vi "HFRR ADV v040 new software.vi"() -> ()   [LabVIEW 2025] (continued)
  # "Move the carriage to the mechanical zero stop — no displacement applied. Before measuring, the sensor must be Preset. Once in position, tap Tare & Begin to zero the reference."
  # "Step 8 — POSITION MEASUREMENT"
  # "Measurement Checklist"
  # "Position the carriage at exactly this \nvalue using your reference gauge, then tap Confirm &\n Next."
  # "Stroked recorded!\n\nTap Confirm & Next  to review the calibration summary."
  # "Step 9 — CALIBRATION RESULT"
  # "Stroke Calibration Complete"
  # "Calibration completed successfully. The measured stroke length is within the acceptable tolerance range of the factory calibration value."
  # "Calibration failed. The measured stroke length differs from the factory calibration value by more than 20%. Please perform the calibration again."
  # "Step 1 — Ball Holder"
  # "Remove the ball holder by loosening and removing the center screw for Friction calibration."
  # "Step 2 — Disc Holder"
  # "Remove the disc holder by loosening and removing the opposing screws. Clean any fluid present in the disc holder."
  # "Step 3 — Calibration Head"
  # "Place the calibration holder in position and securely tighten the center screw."
  # "Step 4 — Calibration Holder"
  # "Place the calibration holder in position and tighten the two securing screws"
  # "Step 5 — Tare (Spring at Free Length)"
  # "Ensure the spring is at its contact (compressed) length — the micrometer head is in contact. Click Tare Sensor to zero the friction force baseline."
  # "Step 6 — Measure Friction Force"
  # "Run the Actual Test to measure Friction Force."
  # "Spring Constant: k = 1.000 N/mm\nSpring force |F| = k Ч d"
  # "Calibrates the ambient air temperature sensor."
  # "Calibrates the sample temperature sensor."
  # "Set B\n60 °C\nHigh-point calibration"
  # "Set A\n0 °C\nIce-point calibration"
  # "Set B\n60 °C\nHigh-point calibration"
  # "Set A\n0 °C\nIce-point calibration"
  # "Select Temperature Sensor"
  # "Choose which temperature sensor you are calibrating. Both use the same two-\npoint procedure: 0 °C (ice-point) and 60 °C (high-point)."
  # "Step 1 — Reference Instrument Setup"
  # "Connect a calibrated reference to the DUT port. This calibration performs two sets: one at 0 °C and one at 60 °C."
  # "Set A\n0 °C\nIce-point calibration"
  # "Set B\n60 °C\nHigh-point calibration"
  # "Allow the temperature bath to stabilise for at least 2 minutes at each set-point before recording the reading."
  # "Step 2 — Set A:  0 °C Calibration"
  # "Connect the  0 °C reference connector. Wait for the temperature to stabilise. Once stable, and click Record Point."
  # "Step 3 — Set A:  60 °C Calibration"
  # "Connect the  60 °C reference connector. Wait for the temperature to stabilise. Once stable, and click Record Point."
  # "Sample Temperature Calibration Complete"
  # "Sample Temperature Calibration PASSED\nMax deviation 0.200 °C — within ±0.5 °C tolerance. Two-point correction applied (0 °C & 60 °C)."
  # "Sample  Temperature Calibration Failed\nmeasured Sample Temperature differs from the factory calibration value"
  # "Step 1 — Reference Instrument Setup"
  # "Connect a calibrated reference to the DUT port. This calibration performs two sets: one at 0 °C and one at 60 °C."
  # "Set A\n0 °C\nIce-point calibration"
  # "Set B\n60 °C\nHigh-point calibration"
  # "Allow the temperature bath to stabilise for at least 2 minutes at each set-point before recording the reading."
  # "Step 2 — Set A:  0 °C Calibration"
  # "Connect the  0 °C reference connector. Wait for the temperature to stabilise. Once stable, and click Record Point."
  # "Step 3 — Set A:  60 °C Calibration"
  # "Connect the  60 °C reference connector. Wait for the temperature to stabilise. Once stable, and click Record Point."
  # "Air Temperature Calibration Complete"
  # "Air Temperature Calibration PASSED\nMax deviation 0.200 °C — within ±0.5 °C tolerance. Two-point correction applied (0 °C & 60 °C)."
  # "Air  Temperature Calibration Failed\nmeasured Sample Temperature differs from the factory calibration value"
  # "System Control Commands\nS;1 - Starts the full automation cycle (Runs Priming-humidify till 70RH sequence first, then switches to Maintenance).\nS;0 - Stops the system immediately and enters Standby mode (Safe State: All actuators OFF).\nM;1 - Skips the priming sequence and jumps directly to Maintenance mode (PID control).\nR;1 - Resets the logic state machine and clears all errors, returning to Standby.\nService Mode (Manual Control)\nX;1 - Enters Manual Service Mode. This disables all automatic logic, sensor safety checks, and timers.\nX;0 - Exits Manual Service Mode and returns to Standby (Safe State).\nActuator Commands (Only work after sending X;1)\nP;[0-255] - Sets the Pump PWM. Note that this is Active Low (0 = Max Flow, 255 = Pump OFF).\nF;I;[0-255] - Sets the Intake Fan speed (0 = OFF, 255 = Max Speed).\nF;O;[0-255] - Sets the Exhaust Fan speed (0 = OFF, 255 = Max Speed).\nD;1 - Turns the Dehumidifier Relay ON.\nD;0 - Turns the Dehumidifier Relay OFF."
  # "%RH"
  # "ISO : WS1.4"
  # "Start test and end test log--- done\nDisable heater ON and Humidity ON during the test --- done\ntemprature and ---done\nhumidity reach log\nauto start run true logic and log\nmanual start log once"
  # "Reference Fluid Information"
  # "Note:\nMake sure to place all images in the folder \"C:\\WinDucom\\im\" before clicking on \"Import Image.\""
  # "NOTE:\nPlace all the images in the path \"C:\\WinDucom\\im\" before clicking on Import Image"
  # "Wear Scar Measurements"
  # "Reference Fluid Information"
  # "Graph :"
types:
  T1 = enum32{"Home", "Dashboard", "Imaging", "Report", "Analysis", "About", "Test Setup", "Advance", "Calibration"}
  T2 = enum32{"HOME", "Test Setup", "Acquire", "Adv Scar", "Adv Scar Report", "Compare Files", "Calibration", "About", "Advance", "Mooha"}
  T3 = enum16{"ASTM D6079", "ISO 12156", "CEC F-096-A-06", "Custom"}
  T4 = enum32{"Dashboard 1", "Dashboard 2", "Dashboard 3"}
  T5 = enum32{"COF", "Friction", "ECR", "Temperature", "Stroke"}
  T6 = enum32{"Coefficient Of Friction", "Air Temperature", "Humidity", "Stroke", "Sample Temperature", "Electrical Contact Resistance", "Frequency", "Air Temp vs Rh"}
  T7 = enum32{"Main", "Stroke", "Friction", "Temperature"}
  T8 = enum32{"Stroke Calibration", "Friction Force Calibration", "Temperature Calibration", "Default"}
  T9 = enum32{"Step 1", "Step 2", "Step 3", "Step 4", "Step 5", "Step 6", "Step 7", "Step 8", "Step 9"}
  T10 = enum32{"Test Progress", "Stroke Points Completed"}
  T11 = enum32{"Page 1", "Page 2", "Page 3", "Page 4", "Page 5", "Page 6", "Page 7"}
  T12 = enum32{"Main", "Step 1", "Step 2", "Step 3", "Step 4", "Air Step 1", "Air Step 2", "Air Step 3", "Air Step 4"}
  T13 = enum32{"Air Temperature", "Sample Temperature", "Default"}
  T14 = enum32{"COMMUNICATION", "CALIBRATION", "Temp Variables", "Camera", "WO 2465 (1)", "WO 2465 (2)", "WO 2465 (3)"}
  T15 = typedef "Auto Start enum.ctl" = enum16{"Init", "Humidity & Temperature On", "Reach point", "Maintain Stage", "Start Stage", "close", "Exit"}
  T16 = typedef "imagedata.ctl" = cluster{"image type":i32, "image depth":i32, "image":u8[], "mask":u8[], "colors":u32[], "Rectangle":cluster{"left":i16, "top":i16, "right":i16, "bottom":i16}}
  T17 = enum32{"HOME", "Test Setup", "Acquire", "Compare Files", "Print Report", "About", "Advance", "Mooha"}
  T18 = cluster{"Read Heave and Surge":string, "Bytes at Heave Port":dbl, "Heave and Surge COM Port:":refnum<visa-resource-name>, "Com Port 2":refnum<visa-resource-name>, "Residual Due":string, "Heave COM Status 2":bool, "Heave COM Status":bool, "Port 2":bool, "Sway PPR":dbl, "Surge PPR":dbl, "Heave PPR":dbl, "Sway Pitch":dbl, "Surge Pitch":dbl, "Heave Pitch":dbl, "Sway Pulses/mm":dbl, "Surge Pulses/mm":dbl, "Heave Pulses/mm":dbl, "inner loop":dbl, "Read Heave and Surge 2":string, "String 36":string, "Write S":bool, "WriteCC1":string[], "Heave COM Loop":i32, "LastCom":string, "EXIT":bool, "Error Heave":errorcluster}
  T19 = enum8{"Enabled", "Disabled", "Disabled and Grayed Out"}
  T20 = cluster{"Read Uno":string, "Bytes at Heave Port":dbl, "UNO COM Port:":refnum<visa-resource-name>, "UNO COM Port: 2":refnum<visa-resource-name>, "Residual Due":string, "UNO COM Status 2":bool, "UNO COM Status":bool, "Port 2":bool, "Sway PPR":dbl, "Surge PPR":dbl, "Heave PPR":dbl, "Sway Pitch":dbl, "Surge Pitch":dbl, "Heave Pitch":dbl, "Sway Pulses/mm":dbl, "Surge Pulses/mm":dbl, "Heave Pulses/mm":dbl, "inner loop":dbl, "Read Heave and Surge 2":string, "String 36":string, "Write S":bool, "WriteCC1":string[], "Heave COM Loop":i32, "LastCom":string, "EXIT":bool, "Error Heave":errorcluster}
  T21 = enum32{"HOME", "Test Setup", "Acquire", "Adv Scar", "Adv Scar Report", "Compare Files", "About", "Advance", "Mooha"}
  T22 = typedef "POST ANALYSIS ENUM.ctl" = enum16{"OPEN EXE", "INIT", "OPEN FILE", "FIT", "DRAW REC", "DRAW LINE", "PAN", "ZOOM IN", "ZOOM OUT", "SET ZOOM", "CLEAR ROI", "GET MEASUREMENTS", "RESIZE MODE", "STREAM START", "STREAM STOP", "SHOW UI", "MINIMIZE UI", "HIDE UI", "CKISE APP", "CLOSE CONNECTION", "SAVE IMAGE", "SET ROI COLOR", "READ", "TCP CHECK", "CLOSE"}
  T23 = typedef "CAMERA LIVE FEED ENUM.ctl" = enum16{"OPEN EXE", "INIT", "READ", "CAMERA CONNECT", "CAMERA START", "CAMERA STOP", "CAMERA GRAY", "CAMERA RGB", "CAMERA MINIMIZE", "CAMERA CLOSE", "CAMERA MODE LIST", "CAMERA MODE SET", "CAMERA RESTORE", "CAMERA SAVE", "CLOSE"}
  T24 = enum16{"Always On", "Always Off", "Off While Running"}
  T25 = enum32{"Page 1", "Page 2", "Page 3", "Page 4", "Page 5", "Page 6"}
  T26 = enum32{"Home", "Dashboard", "Imaging", "Report", "Analysis", "About", "Test Setup", "Advance"}
  T27 = cluster{"File Name":string, "Test Method":string, "Operator":string, "Fuel Description":string, "Date and time":string}
  T28 = enum32{"Home", "Dashboard", "Imaging", "Report", "Analysis", "About", "Test Setup"}
  T29 = enum32{"HOME", "Test Setup", "Acquire", "Compare Files", "About", "Advance", "Mooha"}
  T30 = typedef "NI_ReportGenerationCore.lvlib/HTML Report Image Alignment.ctl" = enum16{"(default)", "LEFT", "RIGHT", "TOP", "TEXTTOP", "MIDDLE", "ABSMIDDLE", "BASELINE", "BOTTOM", "ABSBOTTOM"}
  T31 = cluster{"y":dbl, "LVDT STROKE DISPLAY":dbl, "y":dbl}
  T32 = enum16{"INIT", "READ", "MANUAL WRITE", "WRITE", "CLOSE", "ERROR INIT"}
diagram:
  w3 = 0.0 ("ch0_filt")
  w5 = -9999999.0 ("max_ch0")
  w6 = 9999999.0 ("min_ch0")
  w17 = FALSE ("Visible")
  w18 = T19."Enabled" ("Disabled")
  w21 = FALSE ("Visible")
  w20 = FALSE ("Humidity Off Command")
  w36 = "" ("USER ID")
  (unwired) T21."HOME" ("Main Tab")
  # "[CH1]    - FF\n[CH2]   - TEMPERATURE\n[CH3]    - Humidity\n[CH4]    - AIR TEMP\n[CH5]\\- Visa Uno\n[CH6] \\- Visa Due\n[CH7]  \\- file path\n[CH8]   - Displacement Gain\n[CHA]   - Stroke Gain\n[CHB]   - Stroke PID Gain\n[CHC]   -Language Selection\n[CHD]   -Power +\n[CHE]   -Power_\n[CHF]   -Heater\n[CHG]   -Humidity Wet\n[CHH]   -Humidity Dry\n[CHI]   -Integral Time \n[CHIJ   -Air intercept\n[CHI]   -Temp Intercept"
  n1 = stacked-sequence {
    frame #0 {
    }
    frame #1 {
      n2 = Wait (ms)(milliseconds to wait=u32 1000) -> ()  [unwired: 1 out]
    }
    frame #2 {
      n3 = local write "Due Write"("CAL;SAVE" ("Command")) -> ()
    }
    frame #3 {
      n4 = Wait (ms)(milliseconds to wait=u32 1000) -> ()  [unwired: 1 out]
    }
    frame #4 {
      n5 = local write "Due Write"("CAL;SAVE" ("Command")) -> ()
    }
    frame #5 {
      n6 = Wait (ms)(milliseconds to wait=u32 1000) -> ()  [unwired: 1 out]
    }
    frame #6 {
      # "CAL;END"
      n7 = local write "Due Write"("CAL;END" ("Command")) -> ()
    }
    frame #7 {
      n8 = Wait (ms)(milliseconds to wait=u32 1000) -> ()  [unwired: 1 out]
    }
    frame #8 {
      # "CAL;END"
      n9 = local write "Due Write"("CAL;END" ("Command")) -> ()
    }
    frame #9 {
    }
  }
  n10 = local write "Cal Password"("" ("Cal Password")) -> ()
  n11 = property on="Auto Start Test" class="Bool (strict)"("Visible"=TRUE) -> ()  [unwired: 2 in, 2 out]
  n12 = property on="FRICVALZ 2" class="Bool (strict)"("DisabledEnum"=w18) -> ()  [unwired: 2 in, 2 out]
  n13 = property on="FRICVALZ 4" class="Bool (strict)"("DisabledEnum"=w18) -> ()  [unwired: 2 in, 2 out]
  n14 = property on="FRICVALZ 3" class="Bool (strict)"("DisabledEnum"=w18) -> ()  [unwired: 2 in, 2 out]
  n15 = property on="About" class="Clust (strict)"("Visible"=FALSE) -> ()  [unwired: 2 in, 2 out]
  n16 = property on="Wrong Password" class="Str"("Visible"=w17) -> ()  [unwired: 2 in, 2 out]
  n17 = property on="Calibration 2" class="TabCtl (strict)"("Visible"=w17) -> ()  [unwired: 2 in, 2 out]
  n18 = local write "SCAR MEASURMENT"(enum32{"Auto Scar", "Manual Scar"}."Manual Scar" ("SCAR MEASURMENT")) -> ()
  n19 = flat-sequence {
    tunnel: [w65] -> w2
    tunnel: [w110] -> w28
    tunnel: w2 -> [w105]
    tunnel: [w111] -> w30
    tunnel: w28 -> [w111]
    tunnel: w30 -> [w171]
    tunnel: [w171] -> w29
    tunnel: w29 -> [w202]
    tunnel: [w202] -> w39
    tunnel: w39 -> [w209]
    tunnel: [w215] -> w27
    tunnel: [w203] -> w26
    tunnel: [w257] -> w1
    tunnel: [w256] -> _
    tunnel: w27 -> [w256]
    tunnel: w26 -> [w257]
    frame #0 {
      n20 = call "CLOSE CONNECTION.vi"("error in (no error)"="error in (no error) 2") -> ("error out"=w70:errorcluster)  [unwired: 10 in]
      n21 = call <vilib>:"Clear Errors.vi"("error in (no error)"=w70) -> ("error out"=w69:errorcluster)  [unwired: 5 in, 1 out]
      n22 = disable-structure shown="Enabled" {
        disable-tunnel: w69 -> [w97 _]
        disable-tunnel: [w96 _] -> w68
        frame Enabled {
          n23 = call <userlib>:"Fit VI window to Largest Dec.vi"("error in (no error)"=w97, "border spacing (2 px)"=1) -> ("error out"=w100:errorcluster, "dup VI Ref"=w104:refnum<vi>)  [unwired: 4 in]
          n24 = invoke on="Invoke Node" class="VI" method="FP.Run-Time Position.Maximized"(reference=w104, error in=w100) -> (error out=w101:errorcluster)  [unwired: 2 in, 3 out]
          n25 = call <vilib>:"Clear Errors.vi"("error in (no error)"=w101) -> ("error out"=w103:errorcluster)  [unwired: 5 in, 1 out]
          n26 = control-ref of="This VI"() -> (w95:refnum<vi>)
          n27 = invoke on="Invoke Node" class="VI" method="Default Vals.Reinit All"(reference=w95, error in=w103) -> (reference out=w99:refnum<vi>, error out=w98:errorcluster)  [unwired: 1 in, 1 out]
          n28 = Close Reference(reference=w99, error in (no error)=w98) -> (error out=w96:errorcluster)
        }
        frame Disabled {
        }
      }
      n29 = call "Stall Data Flow.vim"("value in"=w68, "milliseconds to wait"=u32 2000) -> ("value out"=w67:errorcluster)  [unwired: 1 out]
      n30 = call "Read Config.vi"("error in (no error)"=w67) -> ("error out"=w65:errorcluster, "STROKE PARAMETERS"=w76:dbl[], "ADC PARAMETERS"=w77:dbl[], "PID  PARAMETERS"=w78:dbl[], "Stroke Calibration"=w75:string)  [unwired: 6 in]
      n31 = Index Array(array=w76) -> (element #1=w93:dbl, element #2=w94:dbl)  [unwired: 2 in]
      n32 = Index Array(array=w77) -> (element #1=w89:dbl, element #2=w90:dbl, element #3=w91:dbl, element #4=w92:dbl)  [unwired: 4 in]
      n33 = Index Array(array=w78) -> (element #1=w80:dbl, element #2=w81:dbl, element #3=w82:dbl, element #4=w83:dbl, element #5=w84:dbl, element #6=w85:dbl, element #7=w86:dbl, element #8=w87:dbl, element #9=w88:dbl)  [unwired: 9 in]
      n34 = local write "milliseconds to wait"(w80) -> ()
      n35 = local write "dt"(w81) -> ()
      n36 = local write "kp"(w82) -> ()
      n37 = local write "ki"(w83) -> ()
      n38 = local write "kd"(w84) -> ()
      n39 = local write "max_step_change"(w85) -> ()
      n40 = local write "max_amplitude"(w86) -> ()
      n41 = local write "min_amplitude"(w87) -> ()
      n42 = local write "startup_cmd"(w88) -> ()
      n43 = local write "VREF"(w89) -> ()
      n44 = local write "ADC_Resolution"(w90) -> ()
      n45 = local write "PIEZO_CAL_FACTOR"(w91) -> ()
      n46 = local write "NORMAL_FORCE"(w92) -> ()
      n47 = local write "STROKE FILTER"(w93) -> ()
      n48 = local write "Add up Stroke"(w94) -> ()
      n49 = Spreadsheet String To Array(delimiter (Tab)=";", format string="", spreadsheet string=w75, array type (2D Dbl)=dbl[] []) -> (array=w79:dbl[])
      n50 = local write "calibration values"(w79) -> ()
    }
    frame #1 {
      n51 = property on="Auto Scar Check" class="Clust (strict)"("Visible"=TRUE) -> ()  [unwired: 2 in, 2 out]
      n52 = property on="Sign In" class="Bool (strict)"("DisabledEnum"=T19."Disabled" ("Disabled")) -> ()  [unwired: 2 in, 2 out]
      n53 = local write "sign in temp"(FALSE ("sign in temp")) -> ()
      n54 = call "dialog box.vi"("Status"="Before starting the test, verify that the microscope cable is connected.", "error in"=w105) -> ("error out"=w110:errorcluster)  [unwired: 8 in]
    }
    frame #2 {
      (unwired) TRUE ("Re-Initialise")
      # "kkkkk"
      # "C:\\Windows\\wndcm_pw_stdED hfrr.txt"
      # "C:\\LAB-IQ NXT"
      # "C:\\LAB-IQ NXT\\wndcm_pw_stdED hfrr.txt"
      # "password file"
      n55 = Current VI's Path() -> (path=w127:path)
      n56 = Strip Path(path=w127) -> (stripped path=w120:path)  [unwired: 1 out]
      n57 = local write "main tab sub"(enum32{"Page 1", "Page 2"}."Page 1" ("main tab sub")) -> ()
      n58 = local write "Main Tab Display"(T4."Dashboard 1" ("Main Tab Display")) -> ()
      n59 = local write "Main Tab"(T2."HOME" ("Main Tab")) -> ()
      n60 = Path To String(path=w120) -> (string=w122:string)
      n61 = Search/Split String(string=w122, search string/char (-)=".exe") -> (match + rest of string=w124:string)  [unwired: 1 in, 2 out]
      n62 = Match True/False String(2:".vi" ("false string"), 3:".exe" ("true string"), 4:w124) -> (0:w121:bool)  [unwired: 1 out]
      n63 = List Folder(path=path "C:/LAB-IQ" ("directory path"), pattern="*.txt") -> (filenames=w133:string[])  [unwired: 2 in, 3 out]
      n64 = case shown="True" w121 {
        tunnel: w120 -> [w142 w144]
        tunnel: [w142 w143] -> w118
        frame False {
        }
        frame True {
          n65 = Strip Path(path=w144) -> (stripped path=w143:path)  [unwired: 1 out]
        }
      }
      n66 = Search 1D Array(1D array=w133, element="wndcm_pw_stdED hfrr.txt") -> (index of element=w136:i32)  [unwired: 1 in]
      n67 = Equal?(x=w136, y=-1) -> (x = y?=w131:bool)
      n68 = Path To String(path=w118) -> (string=→"Gain path":string)
      n69 = case shown="True" w131 {
        frame False {
        }
        frame True {
          n70 = String To Byte Array(string="123\n") -> (unsigned byte array=w149:u8[])
          n71 = Array Size(array=w149) -> (size(s)=w148:i32)
          n72 = for {
            N: w148 -> [_]
            tunnel: w149 -> [w162]
            tunnel: [w159] -> w151 mode=indexing
            tunnel: w148 -> [w154]
            i -> [w152]
            n73 = Decrement(x=w154) -> (x-1=w155:i32)
            n74 = Index Array(array=w162, index=w152) -> (element=w161:u8)
            n75 = Equal?(x=w152, y=w155) -> (x = y?=w156:bool)
            n76 = Number To Decimal String(number=w161) -> (decimal integer string=w160:string)  [unwired: 1 in]
            n77 = Select(t="", s=w156, f="\r") -> (s? t:f=w153:string)
            n78 = Concatenate Strings(w160, w153) -> (w159:string)
          }
          n79 = local read "file path"() -> (w145:path)
          n80 = Concatenate Strings(w151) -> (w147:string)
          n81 = call <vilib>:"Write Characters To File.vi"("append to file? (new file:F)"=FALSE, "character string"=w147, "file path (dialog if empty)"=w145) -> ()  [unwired: 2 in, 1 out]
        }
      }
      n82 = local write "conststatus"(0.0 ("rpm value : 2")) -> ()
      n83 = local write "EVENT LOG"("") -> ()
      n84 = local write "COUNT"(0 ("COUNT")) -> ()
      n85 = local write "clk"(0.0 ("clk")) -> ()
      n86 = local write "Flag"(0.0 ("Flag")) -> ()
      n87 = local write "Lan flag"(0.0 ("Lan flag")) -> ()
      n88 = local write "Com flag"(u32 0 ("Com flag")) -> ()
      n89 = local write "refresh flag"(FALSE ("refresh flag")) -> ()
      "file path" <- path "C:/LAB-IQ/wndcm_pw_stdED hfrr.txt" ("file path")
      "FF buffer" <- dbl[] [] ("FF buffer")
    }
    frame #3 {
      # "C:\\WinDucom\\calibrate WO 2391.dcf"
      n90 = String To Path(string="C:\\LAB-IQ\\Image Calibrate v01.dcf") -> (path=w166:path)
      n91 = String To Path(string="C:\\LAB-IQ\\calibrate WO 2465.dcf") -> (path=w170:path)
      n92 = Open/Create/Replace File "Open File"(file path (use dialog)=w170) -> (refnum out=w169:refnum<file>)  [unwired: 5 in, 2 out]
      n93 = Open/Create/Replace File ("Open File")(file path (use dialog)=w166) -> (refnum out=w165:refnum<file>)  [unwired: 5 in, 2 out]
      n94 = for {
        N: 4 -> [_]
        tunnel: w165 -> [w177]
        i -> [w173]
        n95 = Read from Text File ("Read File")(file (use dialog)=w177) -> (text=w178:string)  [unwired: 3 in, 3 out]
        n96 = String Subset(string=w178, offset (0)=6, length (rest)=10 ("length (rest)")) -> (substring=w174:string)
        n97 = Fract/Exp String To Number(string=w174) -> (number=w172:dbl)  [unwired: 3 in, 1 out]
        n98 = case shown="3" w173 {
          tunnel: w172 -> [w179 w180 _ w181 _]
          frame 0 {
            n99 = local write "5x Gain"(w179) -> ()
          }
          frame 1 {
            n100 = local write "10x Gain"(w180) -> ()
          }
          frame 2 {
          }
          frame 3 {
            n101 = local write "100x gain"(w181) -> ()
          }
          frame 4, Default {
          }
        }
      }
      n102 = for {
        N: 24 -> [_]
        tunnel: w169 -> [w190]
        i -> [w184]
        (unwired) TRUE ("line mode (F)")
        n103 = Read from Text File "Read File"(file (use dialog)=w190) -> (text=w189:string)  [unwired: 3 in, 3 out]
        n104 = Match Pattern(string=w189, regular expression="]") -> (after substring=w187:string)  [unwired: 1 in, 3 out]
        n105 = String Subset(string=w189, offset (0)=5, length (rest)=10 ("length (rest)")) -> (substring=w182:string)
        n106 = Fract/Exp String To Number(string=w182) -> (number=w183:dbl)  [unwired: 3 in, 1 out]
        n107 = Match Pattern(string=w187, regular expression="-") -> (before substring=w185:string)  [unwired: 1 in, 3 out]
        n108 = case shown="18" w184 {
          tunnel: w183 -> [_ _ _ _ _ _ _ _ _ _ w197 _ _ _ _ _ _ _ _ _ _ _ _ _ _]
          tunnel: w185 -> [_ _ _ _ w193 w194 w195 _ _ _ _ _ _ _ _ _ _ _ _ _ w198 _ w199 w200 _]
          frame 0 {
          }
          frame 1 {
          }
          frame 2 {
          }
          frame 3 {
          }
          frame 4 {
            n109 = local write "Com Port 1"(w193) -> ()
          }
          frame 5 {
            n110 = local write "Com Port 2"(w194) -> ()
            n111 = local write "visa due"(w194) -> ()
          }
          frame 6 {
            n112 = String To Path(string=w195) -> (path=w196:path)
            n113 = local write "File Path"(w196) -> ()
          }
          frame 7 {
          }
          frame 8 {
          }
          frame 9 {
          }
          frame 10 {
            n114 = local write "Language Selection"(w197) -> ()
          }
          frame 11 {
          }
          frame 12 {
          }
          frame 13 {
          }
          frame 14 {
          }
          frame 15 {
          }
          frame 16 {
          }
          frame 17 {
          }
          frame 18 {
          }
          frame 21 {
          }
          frame 22 {
            n115 = local write "Com Port 3"(w198) -> ()
          }
          frame 23 {
          }
          frame 19 {
            n116 = local write "C3 :"(w199) -> ()
          }
          frame 20 {
            n117 = local write "Camera Port :"(w200) -> ()
          }
          frame 24, Default {
          }
        }
      }
    }
    frame #4 {
      n118 = Wait (ms)(milliseconds to wait=u32 1000) -> ()  [unwired: 1 out]
    }
    frame #5 {
      w218 = u32 2000 ("milliseconds to wait")
      w245 = u32 2000 ("milliseconds to wait")
      n119 = call "CAMERA LIVE FEED FGV.vi"("Enum - Menu"=CAMERA_LIVE_FEED_ENUM."OPEN EXE", "error in (no error)"=w209) -> ("error out"=w251:errorcluster)  [unwired: 8 in, 1 out]
      n120 = call "IMAGE ANALYSIS.vi"("Enum"=POST_ANALYSIS_ENUM."OPEN EXE", "error in"=w209) -> ("error out"=w206:errorcluster)  [unwired: 8 in, 1 out]
      n121 = call "Stall Data Flow.vim"("value in"=w251, "milliseconds to wait"=w245) -> ("value out"=w249:errorcluster)  [unwired: 1 out]
      n122 = call "Stall Data Flow.vim"("value in"=w206, "milliseconds to wait"=u32 8000) -> ("value out"=w205:errorcluster)  [unwired: 1 out]
      n123 = call "CAMERA LIVE FEED FGV.vi"("Enum - Menu"=CAMERA_LIVE_FEED_ENUM."INIT", "error in (no error)"=w249) -> ("error out"=w247:errorcluster)  [unwired: 8 in, 1 out]
      n124 = call "IMAGE ANALYSIS.vi"("Enum"=POST_ANALYSIS_ENUM."INIT", "error in"=w205) -> ("error out"=w203:errorcluster)  [unwired: 8 in, 1 out]
      n125 = case shown="Error .." w247 {
        selector: w247 -> [w252 _]
        tunnel: [w252 _] -> w246
        frame No Error {
        }
        frame Error {
          n126 = One Button Dialog(message="Camera initialization error.\nPlease Restart the software") -> ()  [unwired: 1 in, 1 out]
        }
      }
      n127 = property on="Camera Port :" class="CmbBox"() -> ("Strings[]"=w243:string[], "Value"=w244:string)  [unwired: 2 in, 2 out]
      n128 = Search 1D Array(1D array=w243, element=w244) -> (index of element=w242:i32)  [unwired: 1 in]
      n129 = Type Cast(type=30, x=w242) -> (*(type *) &x=w240:i32)
      n130 = call "Stall Data Flow.vim"("value in"=w246, "milliseconds to wait"=w245) -> ("value out"=w222:errorcluster)  [unwired: 1 out]
      n131 = Add(x=w240, y=48) -> (x+y=w221:i32)
      n132 = call "CAMERA LIVE FEED FGV.vi"("Enum - Menu"=CAMERA_LIVE_FEED_ENUM."CAMERA CONNECT", "error in (no error)"=w222, "CAMERA PORT"=w221) -> ("error out"=w231:errorcluster)  [unwired: 7 in, 1 out]
      n133 = call "Stall Data Flow.vim"("value in"=w231, "milliseconds to wait"=u32 5000) -> ("value out"=w232:errorcluster)  [unwired: 1 out]
      n134 = call "CAMERA LIVE FEED FGV.vi"("Enum - Menu"=CAMERA_LIVE_FEED_ENUM."CAMERA MODE LIST", "error in (no error)"=w232) -> ("error out"=w234:errorcluster)  [unwired: 8 in, 1 out]
      n135 = call "Stall Data Flow.vim"("value in"=w234, "milliseconds to wait"=w218) -> ("value out"=w233:errorcluster)  [unwired: 1 out]
      n136 = call "CAMERA LIVE FEED FGV.vi"("Enum - Menu"=CAMERA_LIVE_FEED_ENUM."READ", "error in (no error)"=w233) -> ("error out"=w220:errorcluster, "data out"=→"Camera List":string)  [unwired: 8 in]
      n137 = Type Cast(type=30, x=0) -> (*(type *) &x=w214:i32)
      n138 = call "Stall Data Flow.vim"("value in"=w220, "milliseconds to wait"=w218) -> ("value out"=w219:errorcluster)  [unwired: 1 out]
      n139 = Add(x=w214, y=48) -> (x+y=w212:i32)
      n140 = call "CAMERA LIVE FEED FGV.vi"("Enum - Menu"=CAMERA_LIVE_FEED_ENUM."CAMERA MODE SET", "error in (no error)"=w219, "CAMERA MODE"=w212) -> ("error out"=w216:errorcluster)  [unwired: 7 in, 1 out]
      n141 = call "Stall Data Flow.vim"("value in"=w216, "milliseconds to wait"=u32 2000) -> ("value out"=w236:errorcluster)  [unwired: 1 out]
      n142 = call "CAMERA LIVE FEED FGV.vi"("Enum - Menu"=CAMERA_LIVE_FEED_ENUM."CAMERA START", "error in (no error)"=w236) -> ("error out"=w237:errorcluster)  [unwired: 8 in, 1 out]
      n143 = call "Stall Data Flow.vim"("value in"=w237, "milliseconds to wait"=u32 1000) -> ("value out"=w238:errorcluster)  [unwired: 1 out]
      n144 = call "CAMERA LIVE FEED FGV.vi"("Enum - Menu"=CAMERA_LIVE_FEED_ENUM."CAMERA MINIMIZE", "error in (no error)"=w238) -> ("error out"=w215:errorcluster)  [unwired: 8 in, 1 out]
    }
    frame #6 {
      n145 = case shown="No Error" w256 {
        frame No Error {
          n146 = property on="Auto Scar Check" class="Clust (strict)"("Visible"=FALSE) -> ()  [unwired: 2 in, 2 out]
        }
        frame Error {
        }
      }
      n147 = property on="Sign In" class="Bool (strict)"("DisabledEnum"=T19."Enabled" ("Disabled")) -> ()  [unwired: 2 in, 2 out]
      n148 = local write "sign in temp"(TRUE ("sign in temp")) -> ()
    }
  }
  n149 = local write "Temperature Off Command"(w20) -> ()
  n150 = local write "Main Dashboard Buttons"(T1."Home" ("Main Dashboard Buttons")) -> ()
  n151 = local write "Humidity Off Command"(w20) -> ()
  n152 = local write "CAMERA ROI MIN TEMP"(w20) -> ()
  n153 = local write "TEST FILE NAM,E SAVED"(w20) -> ()
  n154 = local write "LIVE FEED MIN TEMP"(w20) -> ()
  n155 = local write "SCAR MEASURMENT"(enum32{"Auto Scar", "Manual Scar"}."Manual Scar" ("SCAR MEASURMENT")) -> ()
  n156 = local write "Auto stop temp"(w21) -> ()
  n157 = local write "main tab sub"(enum32{"Page 1", "Page 2"}."Page 1" ("main tab sub")) -> ()
  n158 = local write "USERNAME"(w36) -> ()
  n159 = local write "Main Tab"(T2."HOME" ("Main Tab")) -> ()
  n160 = local write "USER ID"(w36) -> ()
  n161 = property on="Auto Scar Check  2" class="Clust (strict)"("Visible"=w21) -> (error out=w24:errorcluster)  [unwired: 2 in, 1 out]
  n162 = property on="Quit" class="Bool (strict)"("Value"=FALSE ("Quit")) -> (error out=w38:errorcluster)  [unwired: 2 in, 1 out]
  n163 = while {
    stop <- w259 stop-if-true
    n164 = event shown="[11] \"Info\": Value Change" {
      selector: _ -> [_ _ _ _ _ _ _ _ _ _ _ _ _ _ _ _ _ _ _ _ _ _ _ _ _ _ _ _ _ _ _ _ _ _ _ _ _ _ _ _ _ _ _ _ _ _ _ _ _ _ _]
      dyn-events: _ -> [_ _ _ _ _ _ _ _ _ _ _ _ _ _ _ _ _ _ _ _ _ _ _ _ _ _ _ _ _ _ _ _ _ _ _ _ _ _ _ _ _ _ _ _ _ _ _ _ _ _ _]
      timeout: 100 -> [_ _ _ _ _ _ _ _ _ _ _ _ _ _ _ _ _ _ _ _ _ _ _ _ _ _ _ _ _ _ _ _ _ _ _ _ _ _ _ _ _ _ _ _ _ _ _ _ _ _ _]
      tunnel: [FALSE FALSE FALSE _ FALSE _ _ _ _ _ _ _ _ _ _ _ _ _ _ _ _ _ _ _ _ _ _ _ _ _ _ _ _ _ _ _ _ _ _ _ _ _ _ _ _ _ _ _ _ _ TRUE] -> w259
      event Timeout {
        n165 = event-data() -> ()  [unwired: 1 in, 3 out]
        n166 = disable-structure shown="Disabled" {
          frame Disabled {
            n167 = local read "Auto Start Test"() -> (w273:bool)
            n168 = local read "RUN"() -> (w274:bool)
            n169 = Or(x=w274, y=w273) -> (x .or. y?=w272:bool)
            n170 = case shown="True" w272 {
              frame False {
                w275 = TRUE ("PAUSE")
                n171 = call "ELAPSED TIMER VI - abort test.vi"("RESET"=w275, "PAUSE"=w275) -> ()  [unwired: 7 in, 3 out]
              }
              frame True {
                n172 = local read "Stroke 2"() -> (w280:dbl)
                n173 = local read "FF 3"() -> (w282:dbl)
                n174 = Equal?(x=w280, y=0.95 ("Stroke 2")) -> (x = y?=w277:bool)
                n175 = Equal?(x=w282, y=0.0 ("FF 3")) -> (x = y?=w278:bool)
                n176 = Or(x=w278, y=w277) -> (x .or. y?=w276:bool)
                n177 = case shown="True" w276 {
                  selector: w276 -> [_ w287]
                  frame False {
                    w283 = TRUE ("PAUSE")
                    n178 = call "ELAPSED TIMER VI - abort test.vi"("RESET"=w283, "PAUSE"=w283) -> ()  [unwired: 7 in, 3 out]
                  }
                  frame True {
                    n179 = Not(x=w287) -> (.not. x?=w286:bool)
                    n180 = call "ELAPSED TIMER VI - abort test.vi"("TARGET"=60.0, "RESET"=w286, "PAUSE"=FALSE) -> ("ELAPSED INDICATION"=w284:bool)  [unwired: 6 in, 2 out]
                    n181 = case shown="True" w284 {
                      frame False {
                      }
                      frame True {
                        n182 = stacked-sequence {
                          frame #0 {
                            w289 = FALSE
                            n183 = local write "RUN"(w289) -> ()
                            n184 = local write "Auto Start Test"(w289) -> ()
                          }
                          frame #1 {
                            n185 = One Button Dialog(message="Test stopped due to a communication error. Reconnect the C1 and C2 cables.") -> ()  [unwired: 1 in, 1 out]
                          }
                        }
                      }
                    }
                  }
                }
              }
            }
          }
          frame Enabled {
          }
        }
        n186 = Get Date/Time In Seconds() -> (seconds since 1Jan1904=w270:timestamp)
        n187 = Format Into String(format string="%<%I:%M:%S:%p %d:%B:%Y>T", w270) -> (resulting string=→"Time Stamp":string)  [unwired: 2 in, 1 out]
        n188 = local read "Service Password enable"() -> (w262:bool)
        n189 = local read "FILE"() -> (w267:string)
        n190 = call <vilib>:"Trim Whitespace.vi"("string"=w267) -> ("trimmed string"=w266:string)  [unwired: 1 in]
        n191 = String Length(string=w266) -> (length=w265:i32)
        n192 = Greater?(x=w265, y=1) -> (0:w263:bool)
        n193 = case shown="False" w263 {
          tunnel: w262 -> [w291 _]
          frame False {
            n194 = case shown="False" w291 {
              frame True {
                w292 = "Test Start In Service Mode" ("Tip Strip")
                w293 = T19."Enabled" ("Disabled")
                n195 = property on="Auto Start Test" class="Bool (strict)"("DisabledEnum"=w293, "TipStrip"=w292) -> ()  [unwired: 2 in, 2 out]
                n196 = property on="RUN" class="Bool (strict)"("DisabledEnum"=w293, "TipStrip"=w292) -> ()  [unwired: 2 in, 2 out]
              }
              frame False {
                w294 = "Enter File Name to Start Test" ("Tip Strip")
                w295 = T19."Disabled and Grayed Out" ("Disabled")
                n197 = property on="Auto Start Test" class="Bool (strict)"("DisabledEnum"=w295, "TipStrip"=w294) -> ()  [unwired: 2 in, 2 out]
                n198 = property on="RUN" class="Bool (strict)"("DisabledEnum"=w295, "TipStrip"=w294) -> ()  [unwired: 2 in, 2 out]
              }
            }
          }
          frame True {
            w296 = "" ("Tip Strip")
            w297 = T19."Enabled" ("Disabled")
            n199 = property on="Auto Start Test" class="Bool (strict)"("DisabledEnum"=w297, "TipStrip"=w296) -> ()  [unwired: 2 in, 2 out]
            n200 = property on="RUN" class="Bool (strict)"("DisabledEnum"=w297, "TipStrip"=w296) -> ()  [unwired: 2 in, 2 out]
          }
        }
      }
      event "RUN": Value Change {
        n201 = event-data() -> ()  [unwired: 1 in, 6 out]
        n202 = local read "RUN"() -> (w299:bool)
        n203 = case shown="False" w299 {
          frame False {
            n204 = flat-sequence {
              frame #0 {
                n205 = local write "START TEMP"(FALSE ("START TEMP")) -> ()
              }
              frame #1 {
                n206 = Wait (ms)(milliseconds to wait=u32 1500) -> ()  [unwired: 1 out]
              }
              frame #2 {
                "HUMIDITY CLEAR" <- TRUE ("HUMIDITY CLEAR")
              }
              frame #3 {
                n207 = local write "Due Write"("VC;0") -> ()
              }
              frame #4 {
                n208 = Wait (ms)(milliseconds to wait=u32 1500) -> ()  [unwired: 1 out]
              }
              frame #5 {
                w309 = T19."Enabled" ("Disabled")
                (unwired) T26."Imaging" ("Main Dashboard Buttons")
                (unwired) T21."Adv Scar" ("Main Tab")
                w311 = "" ("FILE")
                n209 = local write "measured_stroke"(0.0 ("measured_stroke")) -> ()
                n210 = local write "Due Write"("VC;0") -> ()
                n211 = local write "FILE"(w311) -> ()
                n212 = local write "Batch Ref Num :"(w311) -> ()
                n213 = local write "Fuel Discription :"(w311) -> ()
                n214 = local write "Main Tab"(T2."Adv Scar" ("Main Tab")) -> ()
                n215 = local write "Remarks :"(w311) -> ()
                n216 = local write "Main Dashboard Buttons"(T1."Imaging" ("Main Dashboard Buttons")) -> ()
                n217 = local write "TEST FILE NAM,E SAVED"(FALSE ("TEST FILE NAM,E SAVED")) -> ()
                n218 = property on="Stroke ( mm )" class="WFChart (strict)"("History Data"=cluster{"y":dbl, dbl, "y":dbl}[] []) -> ()  [unwired: 2 in, 2 out]
                n219 = property on="Auto Start Test" class="Bool (strict)"("Visible"=TRUE) -> ()  [unwired: 2 in, 2 out]
                n220 = property on="FRICVALZ 2" class="Bool (strict)"("DisabledEnum"=w309) -> ()  [unwired: 2 in, 2 out]
                n221 = property on="FRICVALZ 4" class="Bool (strict)"("DisabledEnum"=w309) -> ()  [unwired: 2 in, 2 out]
                n222 = property on="FRICVALZ 3" class="Bool (strict)"("DisabledEnum"=w309) -> ()  [unwired: 2 in, 2 out]
              }
            }
          }
          frame True {
            n223 = stacked-sequence {
              frame #0 {
                n224 = local write "Due Write"("DAC;200") -> ()
              }
              frame #1 {
                n225 = Wait (ms)(milliseconds to wait=u32 1500) -> ()  [unwired: 1 out]
              }
              frame #2 {
                n226 = local write "Due Write"("DAC;200") -> ()
              }
              frame #3 {
                n227 = Wait (ms)(milliseconds to wait=u32 1500) -> ()  [unwired: 1 out]
              }
              frame #4 {
                n228 = local write "Due Write"("VC;1") -> ()
              }
              frame #5 {
                n229 = Wait (ms)(milliseconds to wait=u32 2000) -> ()  [unwired: 1 out]
              }
              frame #6 {
                n230 = local write "Due Write"("VC;1") -> ()
              }
              frame #7 {
                n231 = Wait (ms)(milliseconds to wait=u32 2000) -> ()  [unwired: 1 out]
              }
              frame #8 {
                w323 = T19."Disabled" ("Disabled")
                n232 = property on="Auto Start Test" class="Bool (strict)"("Visible"=FALSE) -> ()  [unwired: 2 in, 2 out]
                n233 = local write "START TEMP"(TRUE ("START TEMP")) -> ()
                n234 = property on="FRICVALZ 2" class="Bool (strict)"("DisabledEnum"=w323) -> ()  [unwired: 2 in, 2 out]
                n235 = property on="FRICVALZ 4" class="Bool (strict)"("DisabledEnum"=w323) -> ()  [unwired: 2 in, 2 out]
                n236 = property on="FRICVALZ 3" class="Bool (strict)"("DisabledEnum"=w323) -> ()  [unwired: 2 in, 2 out]
              }
            }
          }
        }
      }
      event "run test Calibration": Value Change {
        n237 = event-data() -> ()  [unwired: 1 in, 6 out]
        n238 = local read "run test Calibration"() -> (w325:bool)
        n239 = case shown="False" w325 {
          frame False {
            n240 = flat-sequence {
              frame #0 {
                n241 = local write "START TEMP"(FALSE ("START TEMP")) -> ()
              }
              frame #1 {
                n242 = Wait (ms)(milliseconds to wait=u32 1500) -> ()  [unwired: 1 out]
              }
              frame #2 {
                n243 = local write "HUMIDITY CLEAR"(TRUE) -> ()
              }
              frame #3 {
                n244 = local write "Due Write"("VC;0") -> ()
              }
              frame #4 {
                n245 = Wait (ms)(milliseconds to wait=u32 1500) -> ()  [unwired: 1 out]
              }
              frame #5 {
                n246 = local write "Due Write"("VC;0") -> ()
              }
            }
          }
          frame True {
            n247 = flat-sequence {
              frame #0 {
                n248 = local write "Due Write"("VC;1") -> ()
              }
              frame #1 {
                n249 = Wait (ms)(milliseconds to wait=u32 2000) -> ()  [unwired: 1 out]
              }
              frame #2 {
                n250 = local write "Due Write"("VC;1") -> ()
              }
              frame #3 {
                n251 = Wait (ms)(milliseconds to wait=u32 2000) -> ()  [unwired: 1 out]
              }
              frame #4 {
                n252 = local write "START TEMP"(TRUE ("START TEMP")) -> ()
              }
            }
          }
        }
      }
      event "Auto": Value Change {
        n253 = event-data() -> ()  [unwired: 1 in, 6 out]
        n254 = stacked-sequence {
          frame #0 {
            n255 = local write "FILE"("") -> ()